vi "SaccadeAnalyser - Main.vi"(8 "error in (no error)":errorcluster, 11 "Data IN":T3={"Impulse Positions"=[{"Start"=5471, "End"=5813, "Impulse Plane"=enum."Yaw", "Impulse Direction +ve?"=FALSE, "Time offset"=0, "Amplitude offset"=0.0}, {"Start"=6974, "End"=7325, "Impulse Plane"=enum."Yaw", "Impulse Direction +ve?"=TRUE, "Time offset"=0, "Amplitude offset"=0.0}, {"Start"=7641, "End"=7980, "Impulse Plane"=enum."Yaw", "Impulse Direction +ve?"=FALSE, "Time offset"=0, "Amplitude offset"=0.0}, {"Start"=9060, "End"=9400, "Impulse Plane"=enum."Yaw", "Impulse Direction +ve?"=FALSE, "Time offset"=0, "Amplitude offset"=0.0}, {"Start"=9938, "End"=10282, "Impulse Plane"=enum."Yaw", "Impulse Direction +ve?"=FALSE, "Time offset"=0, "Amplitude offset"=0.0}, {"Start"=10800, "End"=11142, "Impulse Plane"=enum."Yaw", "Impulse Direction +ve?"=FALSE, "Time offset"=0, "Amplitude offset"=0.0}, {"Start"=11602, "End"=11942, "Impulse Plane"=enum."Yaw", "Impulse Direction +ve?"=TRUE, "Time offset"=0, "Amplitude offset"=0.0}, {"Start"=12449, "End"=12790, "Impulse Plane"=enum."Yaw", "Impulse Direction +ve?"=TRUE, "Time offset"=0, "Amplitude offset"=0.0}, {"Start"=13310, "End"=13653, "Impulse Plane"=enum."Yaw", "Impulse Direction +ve?"=TRUE, "Time offset"=0, "Amplitude offset"=0.0}, {"Start"=14191, "End"=14535, "Impulse Plane"=enum."Yaw", "Impulse Direction +ve?"=TRUE, "Time offset"=0, "Amplitude offset"=0.0}, {"Start"=15040, "End"=15380, "Impulse Plane"=enum."Yaw", "Impulse Direction +ve?"=FALSE, "Time offset"=0, "Amplitude offset"=0.0}, {"Start"=16780, "End"=17124, "Impulse Plane"=enum."Yaw", "Impulse Direction +ve?"=TRUE, "Time offset"=0, "Amplitude offset"=0.0}, {"Start"=17572, "End"=17913, "Impulse Plane"=enum."Yaw", "Impulse Direction +ve?"=FALSE, "Time offset"=0, "Amplitude offset"=0.0}, {"Start"=18369, "End"=18713, "Impulse Plane"=enum."Yaw", "Impulse Direction +ve?"=FALSE, "Time offset"=0, "Amplitude offset"=0.0}, {"Start"=19174, "End"=19519, "Impulse Plane"=enum."Yaw", "Impulse Direction +ve?"=FALSE, "Time offset"=0, "Amplitude offset"=0.0}, {"Start"=19928, "End"=20270, "Impulse Plane"=enum."Yaw", "Impulse Direction +ve?"=TRUE, "Time offset"=0, "Amplitude offset"=0.0}, {"Start"=20762, "End"=21121, "Impulse Plane"=enum."Yaw", "Impulse Direction +ve?"=FALSE, "Time offset"=0, "Amplitude offset"=0.0}, {"Start"=21554, "End"=21888, "Impulse Plane"=enum."Yaw", "Impulse Direction +ve?"=FALSE, "Time offset"=0, "Amplitude offset"=0.0}, {"Start"=22293, "End"=22639, "Impulse Plane"=enum."Yaw", "Impulse Direction +ve?"=TRUE, "Time offset"=0, "Amplitude offset"=0.0}, {"Start"=23109, "End"=23464, "Impulse Plane"=enum."Yaw", "Impulse Direction +ve?"=TRUE, "Time offset"=0, "Amplitude offset"=0.0}, {"Start"=23868, "End"=24215, "Impulse Plane"=enum."Yaw", "Impulse Direction +ve?"=TRUE, "Time offset"=0, "Amplitude offset"=0.0}, {"Start"=24643, "End"=24992, "Impulse Plane"=enum."Yaw", "Impulse Direction +ve?"=FALSE, "Time offset"=0, "Amplitude offset"=0.0}, {"Start"=25685, "End"=26023, "Impulse Plane"=enum."Yaw", "Impulse Direction +ve?"=FALSE, "Time offset"=0, "Amplitude offset"=0.0}, {"Start"=26431, "End"=26768, "Impulse Plane"=enum."Yaw", "Impulse Direction +ve?"=FALSE, "Time offset"=0, "Amplitude offset"=0.0}, {"Start"=27251, "End"=27595, "Impulse Plane"=enum."Yaw", "Impulse Direction +ve?"=FALSE, "Time offset"=0, "Amplitude offset"=0.0}, {"Start"=28832, "End"=29180, "Impulse Plane"=enum."Yaw", "Impulse Direction +ve?"=TRUE, "Time offset"=0, "Amplitude offset"=0.0}, {"Start"=31028, "End"=31383, "Impulse Plane"=enum."LARP", "Impulse Direction +ve?"=FALSE, "Time offset"=0, "Amplitude offset"=0.0}, {"Start"=32603, "End"=32936, "Impulse Plane"=enum."LARP", "Impulse Direction +ve?"=TRUE, "Time offset"=0, "Amplitude offset"=0.0}, {"Start"=33445, "End"=33779, "Impulse Plane"=enum."LARP", "Impulse Direction +ve?"=TRUE, "Time offset"=0, "Amplitude offset"=0.0}, {"Start"=34276, "End"=34629, "Impulse Plane"=enum."LARP", "Impulse Direction +ve?"=FALSE, "Time offset"=0, "Amplitude offset"=0.0}, {"Start"=35114, "End"=35460, "Impulse Plane"=enum."LARP", "Impulse Direction +ve?"=FALSE, "Time offset"=0, "Amplitude offset"=0.0}, {"Start"=35981, "End"=36324, "Impulse Plane"=enum."LARP", "Impulse Direction +ve?"=TRUE, "Time offset"=0, "Amplitude offset"=0.0}, {"Start"=36920, "End"=37249, "Impulse Plane"=enum."LARP", "Impulse Direction +ve?"=TRUE, "Time offset"=0, "Amplitude offset"=0.0}, {"Start"=37988, "End"=38322, "Impulse Plane"=enum."LARP", "Impulse Direction +ve?"=TRUE, "Time offset"=0, "Amplitude offset"=0.0}, {"Start"=38964, "End"=39324, "Impulse Plane"=enum."LARP", "Impulse Direction +ve?"=FALSE, "Time offset"=0, "Amplitude offset"=0.0}, {"Start"=39948, "End"=40284, "Impulse Plane"=enum."LARP", "Impulse Direction +ve?"=TRUE, "Time offset"=0, "Amplitude offset"=0.0}, {"Start"=40958, "End"=41293, "Impulse Plane"=enum."LARP", "Impulse Direction +ve?"=TRUE, "Time offset"=0, "Amplitude offset"=0.0}, {"Start"=41899, "End"=42229, "Impulse Plane"=enum."LARP", "Impulse Direction +ve?"=TRUE, "Time offset"=0, "Amplitude offset"=0.0}, {"Start"=42801, "End"=43154, "Impulse Plane"=enum."LARP", "Impulse Direction +ve?"=FALSE, "Time offset"=0, "Amplitude offset"=0.0}, {"Start"=43641, "End"=43980, "Impulse Plane"=enum."LARP", "Impulse Direction +ve?"=TRUE, "Time offset"=0, "Amplitude offset"=0.0}, {"Start"=44466, "End"=44821, "Impulse Plane"=enum."LARP", "Impulse Direction +ve?"=FALSE, "Time offset"=0, "Amplitude offset"=0.0}, {"Start"=45388, "End"=45722, "Impulse Plane"=enum."LARP", "Impulse Direction +ve?"=TRUE, "Time offset"=0, "Amplitude offset"=0.0}, {"Start"=46149, "End"=46510, "Impulse Plane"=enum."LARP", "Impulse Direction +ve?"=FALSE, "Time offset"=0, "Amplitude offset"=0.0}, {"Start"=47874, "End"=48206, "Impulse Plane"=enum."LARP", "Impulse Direction +ve?"=TRUE, "Time offset"=0, "Amplitude offset"=0.0}, {"Start"=50143, "End"=50479, "Impulse Plane"=enum."RALP", "Impulse Direction +ve?"=TRUE, "Time offset"=0, "Amplitude offset"=0.0}, {"Start"=50976, "End"=51310, "Impulse Plane"=enum."RALP", "Impulse Direction +ve?"=FALSE, "Time offset"=0, "Amplitude offset"=0.0}, {"Start"=51892, "End"=52226, "Impulse Plane"=enum."RALP", "Impulse Direction +ve?"=FALSE, "Time offset"=0, "Amplitude offset"=0.0}, {"Start"=52839, "End"=53171, "Impulse Plane"=enum."RALP", "Impulse Direction +ve?"=FALSE, "Time offset"=0, "Amplitude offset"=0.0}, {"Start"=53676, "End"=54012, "Impulse Plane"=enum."RALP", "Impulse Direction +ve?"=TRUE, "Time offset"=0, "Amplitude offset"=0.0}, {"Start"=54530, "End"=54877, "Impulse Plane"=enum."RALP", "Impulse Direction +ve?"=FALSE, "Time offset"=0, "Amplitude offset"=0.0}, {"Start"=55371, "End"=55711, "Impulse Plane"=enum."RALP", "Impulse Direction +ve?"=TRUE, "Time offset"=0, "Amplitude offset"=0.0}, {"Start"=56153, "End"=56482, "Impulse Plane"=enum."RALP", "Impulse Direction +ve?"=FALSE, "Time offset"=0, "Amplitude offset"=0.0}, {"Start"=57053, "End"=57390, "Impulse Plane"=enum."RALP", "Impulse Direction +ve?"=FALSE, "Time offset"=0, "Amplitude offset"=0.0}, {"Start"=57954, "End"=58292, "Impulse Plane"=enum."RALP", "Impulse Direction +ve?"=FALSE, "Time offset"=0, "Amplitude offset"=0.0}, {"Start"=58794, "End"=59130, "Impulse Plane"=enum."RALP", "Impulse Direction +ve?"=TRUE, "Time offset"=0, "Amplitude offset"=0.0}, {"Start"=59587, "End"=59931, "Impulse Plane"=enum."RALP", "Impulse Direction +ve?"=TRUE, "Time offset"=0, "Amplitude offset"=0.0}, {"Start"=60399, "End"=60744, "Impulse Plane"=enum."RALP", "Impulse Direction +ve?"=FALSE, "Time offset"=0, "Amplitude offset"=0.0}, {"Start"=61218, "End"=61559, "Impulse Plane"=enum."RALP", "Impulse Direction +ve?"=FALSE, "Time offset"=0, "Amplitude offset"=0.0}, {"Start"=62100, "End"=62442, "Impulse Plane"=enum."RALP", "Impulse Direction +ve?"=FALSE, "Time offset"=0, "Amplitude offset"=0.0}, {"Start"=62989, "End"=63322, "Impulse Plane"=enum."RALP", "Impulse Direction +ve?"=FALSE, "Time offset"=0, "Amplitude offset"=0.0}, {"Start"=63787, "End"=64136, "Impulse Plane"=enum."RALP", "Impulse Direction +ve?"=TRUE, "Time offset"=0, "Amplitude offset"=0.0}, {"Start"=64603, "End"=64953, "Impulse Plane"=enum."RALP", "Impulse Direction +ve?"=FALSE, "Time offset"=0, "Amplitude offset"=0.0}, {"Start"=65462, "End"=65795, "Impulse Plane"=enum."RALP", "Impulse Direction +ve?"=FALSE, "Time offset"=0, "Amplitude offset"=0.0}, {"Start"=66308, "End"=66645, "Impulse Plane"=enum."RALP", "Impulse Direction +ve?"=FALSE, "Time offset"=0, "Amplitude offset"=0.0}, {"Start"=67052, "End"=67402, "Impulse Plane"=enum."RALP", "Impulse Direction +ve?"=TRUE, "Time offset"=0, "Amplitude offset"=0.0}], "No. Imp"=15, "Parameter Time Series"=[{"time offset"=0.0, "Offset"=0.0, "Gain"=1.0, "inverse"=FALSE, "filter data"=FALSE, "dots"=FALSE, "interpolate"=FALSE, "List 1"=5, "Color Box"=6618880, "Boolean"=TRUE}, {"time offset"=0.0, "Offset"=0.0, "Gain"=1.0, "inverse"=FALSE, "filter data"=FALSE, "dots"=FALSE, "interpolate"=FALSE, "List 1"=6, "Color Box"=6618880, "Boolean"=FALSE}, {"time offset"=0.0, "Offset"=0.0, "Gain"=1.0, "inverse"=FALSE, "filter data"=FALSE, "dots"=FALSE, "interpolate"=FALSE, "List 1"=7, "Color Box"=6618880, "Boolean"=FALSE}, {"time offset"=0.0, "Offset"=0.0, "Gain"=1.0, "inverse"=FALSE, "filter data"=FALSE, "dots"=FALSE, "interpolate"=FALSE, "List 1"=13, "Color Box"=16777224, "Boolean"=TRUE}, {"time offset"=0.0, "Offset"=0.0, "Gain"=1.0, "inverse"=FALSE, "filter data"=FALSE, "dots"=FALSE, "interpolate"=FALSE, "List 1"=14, "Color Box"=16777224, "Boolean"=FALSE}, {"time offset"=0.0, "Offset"=0.0, "Gain"=1.0, "inverse"=FALSE, "filter data"=FALSE, "dots"=FALSE, "interpolate"=FALSE, "List 1"=15, "Color Box"=16777224, "Boolean"=FALSE}], "Parameter Impuls Series"=[{"Color"=6618880, "Visible"=TRUE, "Channel"=1, "Invert"=FALSE, "Desaccade"=FALSE, "Offset"=0.0, "Gain"=1.0}, {"Color"=6618880, "Visible"=FALSE, "Channel"=6, "Invert"=FALSE, "Desaccade"=FALSE, "Offset"=0.0, "Gain"=1.0}, {"Color"=6618880, "Visible"=FALSE, "Channel"=7, "Invert"=FALSE, "Desaccade"=FALSE, "Offset"=0.0, "Gain"=1.0}, {"Color"=16777224, "Visible"=TRUE, "Channel"=13, "Invert"=FALSE, "Desaccade"=FALSE, "Offset"=0.0, "Gain"=1.0}, {"Color"=16777224, "Visible"=FALSE, "Channel"=14, "Invert"=FALSE, "Desaccade"=FALSE, "Offset"=0.0, "Gain"=1.0}, {"Color"=16777224, "Visible"=FALSE, "Channel"=15, "Invert"=FALSE, "Desaccade"=FALSE, "Offset"=0.0, "Gain"=1.0}], "Experiment Parameters"={"Freq"=0.0, "Vel"=0, "Acc"=0, "Stimulus"="Head Impulse"}, "Autosort File"=refnum, "Data File"={"Data Channels"=array34x71049[2415666 elements], "Sample Rate"=500, "Channel List"=["Hz Position-in-Head", "Hz Velocity-in-Head", "Hy Position-in-Head", "Hy Velocity-in-Head", "Hx Position-in-Head", "Hx Velocity-in-Head", "Hl Velocity-in-Head", "Hr Velocity-in-Head", "Lx Position-in-Head", "Ly Position-in-Head", "Lz Position-in-Head", "Lx Velocity-in-Head", "Ly Velocity-in-Head", "Lz Velocity-in-Head", "Ll Velocity-in-Head", "Lr Velocity-in-Head", "Rx Position-in-Head", "Ry Position-in-Head", "Rz Position-in-Head", "Rx Velocity-in-Head", "Ry Velocity-in-Head", "Rz Velocity-in-Head", "Rl Velocity-in-Head", "Rr Velocity-in-Head", "Target on/off", "aux input 1", "aux input 2", " ", "", "", "", "Target Hor", "Target Ver", ""]}, "Experiment data path"=path "C:/Users/w.figtree/Desktop/Coils Data/3", "Image data path"=path "/Macintosh HD/Users/patrick/Studium/Diploma Thesis/Data Analysis", "LVS data path"=path "/Macintosh HD/Users/patrick/Studium/Diploma Thesis/Data Analysis", "Raw copy path"=path "/Macintosh HD/Users/patrick/Studium/Diploma Thesis/Data Analysis", "filename"="passive_lvs.lvs", "desaccading parameters"={"Tolerance"=3, "Acc Range"=7000.0, "Sample Rate"=500, "Impulse Plane 2"=enum."Yaw", "Impulse dir"=FALSE}, "Experiment Parameters 2"={"Subject"="SE Trial Short Term", "Strain"="", "Rotation plane"="", "Experimenter"=" ", "Trial"=0.0, "Time"=0.0}, "Excel"={"Excel._Application"=refnum, "Use Excel"=TRUE, "Worksheet SINE"=refnum, "Row SINE"=0, "Worksheet TRANS"=refnum, "Row TRANS"=0}, "Session Config File"=refnum, "Autosort Parameter Set"=4, "EMA Version"="EMA 2016a", "desacc "={"Threshold 1 [Acc]"=7000.0, "Threshold 2 [% of TH1]"=60, "tolerance"=3, "Search WD "=0.1, " always use TH2"=FALSE, "Range"=3.0, "Max time"=120.0, "Min time"=20.0, "Velocity Threshold"=150}, "Cycle Nr for Saccades"={"POS"=0, "NEG"=0}, "calibration name"="u_calibration_1_p00001s001_calib.mat", "Excel"=refnum} {"Parameter Time Series"."time offset" format="%.3f"; "Parameter Time Series"."Gain" format="%.1f"; "Parameter Time Series"."Offset" format="%.1f"; "Parameter Time Series"."List 1" items=["Motor-Pos", "Motor-Vel", "Lx Position-in-Head", "Ly Position-in-Head", "Lz Position-in-Head", "Lx Velocity-in-Head", "Ly Velocity-in-Head", "Lz Velocity-in-Head", "Ll Velocity-in-Head", "Lr Velocity-in-Head", "Lx Accel-in-Head", "Ly Accel-in-Head", "Lz Accel-in-Head", "Rx Position-in-Head", "Ry Position-in-Head", "Rz Position-in-Head", "Rx Velocity-in-Head", "Ry Velocity-in-Head", "Rz Velocity-in-Head", "Rl Velocity-in-Head", "Rr Velocity-in-Head", "Rx Accel-in-Head", "Ry Accel-in-Head", "Rz Accel-in-Head", "Global Trigger", "", "", ""]; "Parameter Impuls Series"."Gain" format="%.1f"; "Parameter Impuls Series"."Offset" format="%.1f"}) -> (0 "error out":errorcluster, 3 "Data OUT":T3={"Impulse Positions"=[{"Start"=5471, "End"=5813, "Impulse Plane"=enum."Yaw", "Impulse Direction +ve?"=FALSE, "Time offset"=0, "Amplitude offset"=0.0}, {"Start"=6974, "End"=7325, "Impulse Plane"=enum."Yaw", "Impulse Direction +ve?"=TRUE, "Time offset"=0, "Amplitude offset"=0.0}, {"Start"=7641, "End"=7980, "Impulse Plane"=enum."Yaw", "Impulse Direction +ve?"=FALSE, "Time offset"=0, "Amplitude offset"=0.0}, {"Start"=9060, "End"=9400, "Impulse Plane"=enum."Yaw", "Impulse Direction +ve?"=FALSE, "Time offset"=0, "Amplitude offset"=0.0}, {"Start"=9938, "End"=10282, "Impulse Plane"=enum."Yaw", "Impulse Direction +ve?"=FALSE, "Time offset"=0, "Amplitude offset"=0.0}, {"Start"=10800, "End"=11142, "Impulse Plane"=enum."Yaw", "Impulse Direction +ve?"=FALSE, "Time offset"=0, "Amplitude offset"=0.0}, {"Start"=11602, "End"=11942, "Impulse Plane"=enum."Yaw", "Impulse Direction +ve?"=TRUE, "Time offset"=0, "Amplitude offset"=0.0}, {"Start"=12449, "End"=12790, "Impulse Plane"=enum."Yaw", "Impulse Direction +ve?"=TRUE, "Time offset"=0, "Amplitude offset"=0.0}, {"Start"=13310, "End"=13653, "Impulse Plane"=enum."Yaw", "Impulse Direction +ve?"=TRUE, "Time offset"=0, "Amplitude offset"=0.0}, {"Start"=14191, "End"=14535, "Impulse Plane"=enum."Yaw", "Impulse Direction +ve?"=TRUE, "Time offset"=0, "Amplitude offset"=0.0}, {"Start"=15040, "End"=15380, "Impulse Plane"=enum."Yaw", "Impulse Direction +ve?"=FALSE, "Time offset"=0, "Amplitude offset"=0.0}, {"Start"=16780, "End"=17124, "Impulse Plane"=enum."Yaw", "Impulse Direction +ve?"=TRUE, "Time offset"=0, "Amplitude offset"=0.0}, {"Start"=17572, "End"=17913, "Impulse Plane"=enum."Yaw", "Impulse Direction +ve?"=FALSE, "Time offset"=0, "Amplitude offset"=0.0}, {"Start"=18369, "End"=18713, "Impulse Plane"=enum."Yaw", "Impulse Direction +ve?"=FALSE, "Time offset"=0, "Amplitude offset"=0.0}, {"Start"=19174, "End"=19519, "Impulse Plane"=enum."Yaw", "Impulse Direction +ve?"=FALSE, "Time offset"=0, "Amplitude offset"=0.0}, {"Start"=19928, "End"=20270, "Impulse Plane"=enum."Yaw", "Impulse Direction +ve?"=TRUE, "Time offset"=0, "Amplitude offset"=0.0}, {"Start"=20762, "End"=21121, "Impulse Plane"=enum."Yaw", "Impulse Direction +ve?"=FALSE, "Time offset"=0, "Amplitude offset"=0.0}, {"Start"=21554, "End"=21888, "Impulse Plane"=enum."Yaw", "Impulse Direction +ve?"=FALSE, "Time offset"=0, "Amplitude offset"=0.0}, {"Start"=22293, "End"=22639, "Impulse Plane"=enum."Yaw", "Impulse Direction +ve?"=TRUE, "Time offset"=0, "Amplitude offset"=0.0}, {"Start"=23109, "End"=23464, "Impulse Plane"=enum."Yaw", "Impulse Direction +ve?"=TRUE, "Time offset"=0, "Amplitude offset"=0.0}, {"Start"=23868, "End"=24215, "Impulse Plane"=enum."Yaw", "Impulse Direction +ve?"=TRUE, "Time offset"=0, "Amplitude offset"=0.0}, {"Start"=24643, "End"=24992, "Impulse Plane"=enum."Yaw", "Impulse Direction +ve?"=FALSE, "Time offset"=0, "Amplitude offset"=0.0}, {"Start"=25685, "End"=26023, "Impulse Plane"=enum."Yaw", "Impulse Direction +ve?"=FALSE, "Time offset"=0, "Amplitude offset"=0.0}, {"Start"=26431, "End"=26768, "Impulse Plane"=enum."Yaw", "Impulse Direction +ve?"=FALSE, "Time offset"=0, "Amplitude offset"=0.0}, {"Start"=27251, "End"=27595, "Impulse Plane"=enum."Yaw", "Impulse Direction +ve?"=FALSE, "Time offset"=0, "Amplitude offset"=0.0}, {"Start"=28832, "End"=29180, "Impulse Plane"=enum."Yaw", "Impulse Direction +ve?"=TRUE, "Time offset"=0, "Amplitude offset"=0.0}, {"Start"=31028, "End"=31383, "Impulse Plane"=enum."LARP", "Impulse Direction +ve?"=FALSE, "Time offset"=0, "Amplitude offset"=0.0}, {"Start"=32603, "End"=32936, "Impulse Plane"=enum."LARP", "Impulse Direction +ve?"=TRUE, "Time offset"=0, "Amplitude offset"=0.0}, {"Start"=33445, "End"=33779, "Impulse Plane"=enum."LARP", "Impulse Direction +ve?"=TRUE, "Time offset"=0, "Amplitude offset"=0.0}, {"Start"=34276, "End"=34629, "Impulse Plane"=enum."LARP", "Impulse Direction +ve?"=FALSE, "Time offset"=0, "Amplitude offset"=0.0}, {"Start"=35114, "End"=35460, "Impulse Plane"=enum."LARP", "Impulse Direction +ve?"=FALSE, "Time offset"=0, "Amplitude offset"=0.0}, {"Start"=35981, "End"=36324, "Impulse Plane"=enum."LARP", "Impulse Direction +ve?"=TRUE, "Time offset"=0, "Amplitude offset"=0.0}, {"Start"=36920, "End"=37249, "Impulse Plane"=enum."LARP", "Impulse Direction +ve?"=TRUE, "Time offset"=0, "Amplitude offset"=0.0}, {"Start"=37988, "End"=38322, "Impulse Plane"=enum."LARP", "Impulse Direction +ve?"=TRUE, "Time offset"=0, "Amplitude offset"=0.0}, {"Start"=38964, "End"=39324, "Impulse Plane"=enum."LARP", "Impulse Direction +ve?"=FALSE, "Time offset"=0, "Amplitude offset"=0.0}, {"Start"=39948, "End"=40284, "Impulse Plane"=enum."LARP", "Impulse Direction +ve?"=TRUE, "Time offset"=0, "Amplitude offset"=0.0}, {"Start"=40958, "End"=41293, "Impulse Plane"=enum."LARP", "Impulse Direction +ve?"=TRUE, "Time offset"=0, "Amplitude offset"=0.0}, {"Start"=41899, "End"=42229, "Impulse Plane"=enum."LARP", "Impulse Direction +ve?"=TRUE, "Time offset"=0, "Amplitude offset"=0.0}, {"Start"=42801, "End"=43154, "Impulse Plane"=enum."LARP", "Impulse Direction +ve?"=FALSE, "Time offset"=0, "Amplitude offset"=0.0}, {"Start"=43641, "End"=43980, "Impulse Plane"=enum."LARP", "Impulse Direction +ve?"=TRUE, "Time offset"=0, "Amplitude offset"=0.0}, {"Start"=44466, "End"=44821, "Impulse Plane"=enum."LARP", "Impulse Direction +ve?"=FALSE, "Time offset"=0, "Amplitude offset"=0.0}, {"Start"=45388, "End"=45722, "Impulse Plane"=enum."LARP", "Impulse Direction +ve?"=TRUE, "Time offset"=0, "Amplitude offset"=0.0}, {"Start"=46149, "End"=46510, "Impulse Plane"=enum."LARP", "Impulse Direction +ve?"=FALSE, "Time offset"=0, "Amplitude offset"=0.0}, {"Start"=47874, "End"=48206, "Impulse Plane"=enum."LARP", "Impulse Direction +ve?"=TRUE, "Time offset"=0, "Amplitude offset"=0.0}, {"Start"=50143, "End"=50479, "Impulse Plane"=enum."RALP", "Impulse Direction +ve?"=TRUE, "Time offset"=0, "Amplitude offset"=0.0}, {"Start"=50976, "End"=51310, "Impulse Plane"=enum."RALP", "Impulse Direction +ve?"=FALSE, "Time offset"=0, "Amplitude offset"=0.0}, {"Start"=51892, "End"=52226, "Impulse Plane"=enum."RALP", "Impulse Direction +ve?"=FALSE, "Time offset"=0, "Amplitude offset"=0.0}, {"Start"=52839, "End"=53171, "Impulse Plane"=enum."RALP", "Impulse Direction +ve?"=FALSE, "Time offset"=0, "Amplitude offset"=0.0}, {"Start"=53676, "End"=54012, "Impulse Plane"=enum."RALP", "Impulse Direction +ve?"=TRUE, "Time offset"=0, "Amplitude offset"=0.0}, {"Start"=54530, "End"=54877, "Impulse Plane"=enum."RALP", "Impulse Direction +ve?"=FALSE, "Time offset"=0, "Amplitude offset"=0.0}, {"Start"=55371, "End"=55711, "Impulse Plane"=enum."RALP", "Impulse Direction +ve?"=TRUE, "Time offset"=0, "Amplitude offset"=0.0}, {"Start" (continued)
104.00000000000001, 106.0, 108.0, 110.0, 112.0, 114.0, 116.0, 118.00000000000001, 120.0, 122.0, 124.0, 126.0, 128.0, 130.0, 132.0, 134.0, 136.0, 138.0, 140.0, 142.00000000000003, 144.00000000000003, 146.0, 148.0, 150.0, 152.0, 154.0, 156.0, 158.0, 160.0, 162.0, 164.0, 166.0, 168.0, 170.0, 172.0, 174.00000000000003, 176.0, 178.0, 180.0, 182.0, 184.0, 186.0, 188.0, 190.0, 192.0, 194.0, 196.0, 198.0, 200.0, 202.0, 204.00000000000003, 206.00000000000003, 208.00000000000003, 210.0, 212.0, 214.0, 216.0, 218.0, 220.0, 222.0, 224.0, 226.0, 228.0, 230.0, 232.0, 234.0, 236.00000000000003, 238.00000000000003, 240.0, 242.0, 244.0, 246.0, 248.0, 250.0, 252.0, 254.0, 256.0, 258.0, 260.0, 262.0, 264.0, 266.0, 268.0, 270.0, 272.0, 274.0, 276.0, 278.0, 280.0, 282.0, 284.00000000000006, 286.00000000000006, 288.00000000000006, 290.0, 292.0, 294.0, 296.0, 298.0, 300.0, 302.0, 304.0, 306.0, 308.0, 310.0, 312.0, 314.0, 316.0, 318.0, 320.0, 322.0, 324.0, 326.0, 328.0, 330.0, 332.0, 334.0, 336.0, 338.0, 340.0, 342.0, 344.0, 346.00000000000006, 348.00000000000006, 350.00000000000006, 352.0, 354.0, 356.0, 358.0, 360.0, 362.0, 364.0, 366.0, 368.0, 370.0, 372.0, 374.0, 376.0, 378.0, 380.0, 382.0, 384.0, 386.0, 388.0, 390.0, 392.0, 394.0, 396.0, 398.0, 400.0, 402.0, 404.0, 406.0, 408.00000000000006, 410.00000000000006, 412.00000000000006, 414.00000000000006, 416.00000000000006, 418.0, 420.0, 422.0, 424.0, 426.0, 428.0, 430.0, 432.0, 434.0, 436.0, 438.0, 440.0, 442.0, 444.0, 446.0, 448.0, 450.0, 452.0, 454.0, 456.0, 458.0, 460.0, 462.0, 464.0, 466.0, 468.0, 470.00000000000006, 472.00000000000006, 474.00000000000006, 476.00000000000006, 478.00000000000006, 480.0, 482.0, 484.0, 486.0, 488.0, 490.0, 492.0, 494.0, 496.0, 498.0, 500.0, 502.0, 504.0, 506.0, 508.0, 510.0, 512.0, 514.0, 516.0, 518.0, 520.0, 522.0, 524.0, 526.0, 528.0, 530.0, 532.0, 534.0, 536.0, 538.0, 540.0, 542.0, 544.0, 546.0, 548.0, 550.0, 552.0, 554.0, 556.0, 558.0, 560.0, 562.0, 564.0, 566.0000000000001, 568.0000000000001, 570.0000000000001, 572.0000000000001, 574.0000000000001, 576.0000000000001, 578.0, 580.0, 582.0, 584.0, 586.0, 588.0, 590.0, 592.0, 594.0, 596.0, 598.0, 600.0, 602.0, 604.0, 606.0, 608.0, 610.0, 612.0, 614.0, 616.0, 618.0, 620.0, 622.0, 624.0, 626.0, 628.0, 630.0, 632.0, 634.0, 636.0, 638.0, 640.0, 642.0, 644.0, 646.0, 648.0, 650.0, 652.0, 654.0, 656.0, 658.0, 660.0, 662.0, 664.0, 666.0, 668.0], [0.04992038201718785, 0.15841417568277905, 0.17858167540149594, 0.15312905238445929, 0.12879273253846435, 0.1386267538312591, 0.19119834871886, 0.26744517118748234, 0.3294694061613903, 0.33604542690323846, 0.26750116445730754, 0.13882756764760273, -0.00457400840335076, -0.08930376240759585, -0.03122544770549318, 0.23626243538025626, 0.7326977878601504, 1.414166028082219, 2.18407302630931, 2.91143092377669, 3.4505976401226643, 3.6807231650130703, 3.538299036917895, 3.0375740961591866, 2.2730290152877277, 1.3923240791589553, 0.572883978458961, -0.015453323814009323, -0.25359029677372646, -0.09697114730811052, 0.41567980525341497, 1.1707413546443597, 2.0010012490946743, 2.7260585284931693, 3.1985829335543183, 3.332956582490871, 3.1222617337603964, 2.63734783762464, 2.0087327672521784, 1.396995356354343, 0.9476382692160676, 0.7553993294950168, 0.8473748527615594, 1.181402058393096, 1.66213162160191, 2.164995642103872, 2.565021706411774, 2.7770579425637756, 2.7777673635849727, 2.6013186150579433, 2.3306813660582852, 2.076819233598228, 1.9481292438628854, 2.016991388073549, 2.2989795669998085, 2.749552100833662, 3.2736328956474297, 3.7499302412652673, 4.060800060130227, 4.125340378912859, 3.9311403507880924, 3.535056197748248, 3.049660186385034, 2.624300893859544, 2.4060875775539285, 2.5093105752294194, 2.993320304677124, 3.848304722717669, 4.996773223397807, 6.318170390599681, 7.688214344644706, 9.003185964170115, 10.196919210919303, 11.260714840565495, 12.2491594060802, 13.258988588333356, 14.398222913355678, 15.763109352234887, 17.41424581629392, 19.365482073801317, 21.586770877674706, 24.015338314877916, 26.582943324362425, 29.244991166590985, 31.999704094019627, 34.89270409467796, 38.013451580925384, 41.4776338903614, 45.39813750442575, 49.86051106407923, 54.8996055102276, 60.487486108843896, 66.54041305150024, 72.92794874389115, 79.49091069527614, 86.0732882383193, 92.54343430335877, 98.81704640232888, 104.86380166453532, 110.69767181947952, 116.36816024047974, 121.93679606634197, 127.44946268816003, 132.91382406412202, 138.29013354077009, 143.49090983609346, 148.39593527181597, 152.87217504466742, 156.79159603077275, 160.06260704130017, 162.64877788792944, 164.5616374633256, 165.8592891901892, 166.6238891626943, 166.93327673497157, 166.84560727192155, 166.3680932814025, 165.45691552757975, 164.02818548071699, 161.96591043080474, 159.16084591883293, 155.5358166070166, 151.06037761889493, 145.77461158069093, 139.7884164622531, 133.25880357201612, 126.36444720474383, 119.2860273986354, 112.17741601561518, 105.1525468650749, 98.28906854847438, 91.62060481380246, 85.14400241893199, 78.84223186193547, 72.69596110254957, 66.67462318862016, 60.74867508111842, 54.90283443323352, 49.126842276315514, 43.417641849534206, 37.78234365969709, 32.24059878511545, 26.836290153038057, 21.634339151746794, 16.701708877871617, 12.103037841181745, 7.896149545815408, 4.1128290788135615, 0.7389662736026011, -2.2694903576020735, -4.9631062834405215, -7.405244086308598, -9.65177273250551, -11.721341930325584, -13.600003955279014, -15.252602221067322, -16.630091323905262, -17.684645898322437, -18.3951576449166, -18.774019507133094, -18.85230364678983, -18.67939872359451, -18.309760473378486, -17.782702973493613, -17.114260366081247, -16.298543546223584, -15.32517813268789, -14.187238566587439, -12.894388212139678, -11.486000357145317, -10.02590465717922, -8.595127553420681, -7.280228618080622, -6.148598180573282, -5.236592749098192, -4.553928778071988, -4.088533383914676, -3.8073230410928036, -3.6630957051259516, -3.6150109657845926, -3.6278390081094547, -3.66903344717268, -3.711385162328716, -3.7175002219534328, -3.638365649322722, -3.4289240476014973, -3.057478585829699, -2.5219742752628402, -1.8586527966781206, -1.1389975609344174, -0.47183019522024927, 0.0051455380020754005, 0.15788917699917693, -0.10050061025888996, -0.7911814548039556, -1.8643562384539165, -3.187405881295393, -4.569498848546866, -5.8139278704619395, -6.7478282463364, -7.253448745420589, -7.307372747595566, -6.984682301078392, -6.435022163171514, -5.849969545435848, -5.425648598324794, -5.325281629094702, -5.63615524890895, -6.352882944462618, -7.384002079740541, -8.559439461424077, -9.668039211518757, -10.503952472324885, -10.908138327541469, -10.803458262192532, -10.209367806756003, -9.24090626674652, -8.080681007005104, -6.944230818795323, -6.037426910342507, -5.506280050693961, -5.404708174170484, -5.685918619423186, -6.21971107762246, -6.82533358689519, -7.309516207965832, -7.517365437937178, -7.366810938149376, -6.847446190723453, -6.027476319138884, -5.037258943036763, -4.021281572243785, -3.106723881663414, -2.3861127603837033, -1.9057193800399248, -1.6641085250296699, -1.6357550842919144, -1.7887182069729657, -2.0797865669803848, -2.4613784430723564, -2.87931328602323, -3.2829278591162554, -3.6399358176747985, -3.930540590692001, -4.185841440412954, -4.519901384583601, -5.112600094423929, -6.179934257207675, -7.911857897301076, -10.380842296632798, -13.456630338729223, -16.750182623917276, -19.63301571121884, -21.335243781207225, -21.081763915218374, -18.2841175327463, -12.734024178915037, -4.708677229533636, 5.018081046184022, 15.273118953586463, 24.69383865631704, 31.990547165492487, 36.19894847480768, 36.8668944349022, 34.13346741147935, 28.680271923098346, 21.551397571814505, 13.9200326044393, 6.853263681311434, 1.109113748113744, -2.9572638183698965, -5.386063683488901, -6.525260094996831, -6.873361693133134, -6.913364973447512, -6.977914337377552, -7.176035360345667, -7.398600739376963, -7.3767525082011804, -6.7782328355304795, -5.314655641339901, -2.8256467063059447, 0.6726090248953283, 4.98148672460113, 9.750320796626117, 14.530187559033408, 18.84255920678958, 22.26067541171979, 24.468305768199688, 25.29294718130975, 24.725614427990152, 22.9030335665933, 20.082655608922238, 16.606151876437476, 12.82963888753322, 9.079726996951507, 5.622531347536689, 2.6217090367480265, 0.13171202491932155, -1.8838458215461478, -3.5233802618856194, -4.91150074028557, -6.173130009585858, -7.408881055173729, -8.664646778406222, -9.92458311171681, -11.12491778059621, -12.164256102990326, -12.926429930262247, -13.308922541262364, -13.239115051984019, -12.688617129803168, -11.680068508276396, -10.28596817566143, -8.619076823723638, -6.8072801732139006, -4.977472566204141, -3.2450998627929843, -1.699500663571817, -0.39723303554407496, 0.6456925599396672, 1.4455339547691926, 2.023868943252673, 2.40182753031554, 2.597658890354133, 2.615611688992259, 2.4512690594426902, 2.097642800762138, 1.5504992618844369, 0.8296317099263332, -0.011760473109973524, -0.898827295135341, -1.7432784721434178, -2.455414534839041]}, {[0.0, 2.0, 4.0, 6.0, 8.0, 10.0, 12.0, 14.0, 16.0, 18.000000000000004, 20.0, 22.0, 24.0, 26.000000000000004, 28.0, 30.0, 32.0, 34.0, 36.00000000000001, 38.0, 40.0, 42.0, 44.0, 46.0, 48.0, 50.0, 52.00000000000001, 54.0, 56.0, 58.0, 60.0, 62.0, 64.0, 66.0, 68.0, 70.0, 72.00000000000001, 74.0, 76.0, 78.0, 80.0, 82.0, 84.0, 86.0, 88.0, 90.0, 92.0, 94.0, 96.0, 98.0, 100.0, 102.00000000000001, 104.00000000000001, 106.0, 108.0, 110.0, 112.0, 114.0, 116.0, 118.00000000000001, 120.0, 122.0, 124.0, 126.0, 128.0, 130.0, 132.0, 134.0, 136.0, 138.0, 140.0, 142.00000000000003, 144.00000000000003, 146.0, 148.0, 150.0, 152.0, 154.0, 156.0, 158.0, 160.0, 162.0, 164.0, 166.0, 168.0, 170.0, 172.0, 174.00000000000003, 176.0, 178.0, 180.0, 182.0, 184.0, 186.0, 188.0, 190.0, 192.0, 194.0, 196.0, 198.0, 200.0, 202.0, 204.00000000000003, 206.00000000000003, 208.00000000000003, 210.0, 212.0, 214.0, 216.0, 218.0, 220.0, 222.0, 224.0, 226.0, 228.0, 230.0, 232.0, 234.0, 236.00000000000003, 238.00000000000003, 240.0, 242.0, 244.0, 246.0, 248.0, 250.0, 252.0, 254.0, 256.0, 258.0, 260.0, 262.0, 264.0, 266.0, 268.0, 270.0, 272.0, 274.0, 276.0, 278.0, 280.0, 282.0, 284.00000000000006, 286.00000000000006, 288.00000000000006, 290.0, 292.0, 294.0, 296.0, 298.0, 300.0, 302.0, 304.0, 306.0, 308.0, 310.0, 312.0, 314.0, 316.0, 318.0, 320.0, 322.0, 324.0, 326.0, 328.0, 330.0, 332.0, 334.0, 336.0, 338.0, 340.0, 342.0, 344.0, 346.00000000000006, 348.00000000000006, 350.00000000000006, 352.0, 354.0, 356.0, 358.0, 360.0, 362.0, 364.0, 366.0, 368.0, 370.0, 372.0, 374.0, 376.0, 378.0, 380.0, 382.0, 384.0, 386.0, 388.0, 390.0, 392.0, 394.0, 396.0, 398.0, 400.0, 402.0, 404.0, 406.0, 408.00000000000006, 410.00000000000006, 412.00000000000006, 414.00000000000006, 416.00000000000006, 418.0, 420.0, 422.0, 424.0, 426.0, 428.0, 430.0, 432.0, 434.0, 436.0, 438.0, 440.0, 442.0, 444.0, 446.0, 448.0, 450.0, 452.0, 454.0, 456.0, 458.0, 460.0, 462.0, 464.0, 466.0, 468.0, 470.00000000000006, 472.00000000000006, 474.00000000000006, 476.00000000000006, 478.00000000000006, 480.0, 482.0, 484.0, 486.0, 488.0, 490.0, 492.0, 494.0, 496.0, 498.0, 500.0, 502.0, 504.0, 506.0, 508.0, 510.0, 512.0, 514.0, 516.0, 518.0, 520.0, 522.0, 524.0, 526.0, 528.0, 530.0, 532.0, 534.0, 536.0, 538.0, 540.0, 542.0, 544.0, 546.0, 548.0, 550.0, 552.0, 554.0, 556.0, 558.0, 560.0, 562.0, 564.0, 566.0000000000001, 568.0000000000001, 570.0000000000001, 572.0000000000001, 574.0000000000001, 576.0000000000001, 578.0, 580.0, 582.0, 584.0, 586.0, 588.0, 590.0, 592.0, 594.0, 596.0, 598.0, 600.0, 602.0, 604.0, 606.0, 608.0, 610.0, 612.0, 614.0, 616.0, 618.0, 620.0, 622.0, 624.0, 626.0, 628.0, 630.0, 632.0, 634.0, 636.0, 638.0, 640.0, 642.0, 644.0, 646.0, 648.0, 650.0, 652.0, 654.0, 656.0, 658.0, 660.0, 662.0, 664.0, 666.0, 668.0], [0.06811297872756228, 0.01707691464348393, -0.0029316795212057656, -0.018371635138466402, -0.0542419341462157, -0.12324447550139972, -0.21981306669672707, -0.3191162631877944, -0.3853854038940563, -0.3843579085985379, -0.30437797985139503, -0.1664789665300923, -0.017769334490307376, 0.06862919302039172, 0.013104685658458237, -0.24114913861073983, -0.709333253854556, -1.351598990540456, -2.075622182814767, -2.753071542994334, -3.246216629685337, -3.443449967376811, -3.286367039037831, -2.791374332901265, -2.051529141203167, -1.2105609505019466, -0.4403291048291216, 0.09601987150864488, 0.28620327185831584, 0.0919344247244478, -0.4423285837620785, -1.1989490655453743, -2.009497024906068, -2.6945611442154345, -3.1102502224856075, -3.1773935367996238, -2.898039897130179, -2.353443274375975, -1.684014162208868, -1.0575586797480234, -0.622984378715925, -0.47347998056239504, -0.6266828095259971, -1.0270679039930393, -1.5690220717276038, -2.1190951404570306, -2.54956813966023, -2.779552448106653, -2.7895908254476565, -2.618860676067743, -2.352435864524903, -2.093848698492252, -1.9367005319072188, -1.9373752595012403, -2.103354399108734, -2.399366287498072, -2.7620015653891814, -3.1211357852220005, -3.4186287524182504, -3.6236871208071846, -3.7450535834045713, -3.817946376182001, -3.8859888168671204, -3.9913068551006026, -4.157735245453354, -4.388591325996881, -4.6732363152460525, -4.994493297578687, -5.337310207009276, -5.702737161776087, -6.121366746488304, -6.643068076473353, -7.320282018360008, -8.205626664881649, -9.342663338610144, -10.751802729833212, -12.428003541980054, -14.3403029147095, -16.440257730359697, -18.674757629156378, -20.993764005443836, -23.36094550703045, -25.766167573394647, -28.235984867149952, -30.83064641351026, -33.63339995706863, -36.745311701228715, -40.27040505521088, -44.29407874919056, -48.870946189857676, -54.00959526902649, -59.663906206975355, -65.7386581494263, -72.09737120363829, -78.58246030020933, -85.0352581421007, -91.3134523513386, -97.31362354068435, -102.97527187162223, -108.28408268059235, -113.26702471639702, -117.96733172180792, -122.42684847414944, -126.66981282582509, -130.68989907667182, -134.44283460888644, -137.85244951870885, -140.82165420094103, -143.24223062902917, -145.02170566485017, -146.1037912555284, -146.46968334697482, -146.1471196893165, -145.20629627467477, -143.74220064879705, -141.85872825081555, -139.64370902034784, -137.15798008041577, -134.42257527977037, -131.4126853108042, -128.08076518877618, -124.36618833100033, -120.20643043471809, -115.56964072369297, -110.4603120398877, -104.91662067262685, -99.01459414696029, -92.84879592980549, -86.51455625875208, -80.10405919393807, -73.69570633615069, -67.34436860943498, -61.079868879950936, -54.91881846904339, -48.8738566758385, -42.94324202006271, -37.12579137611928, -31.43575468987897, -25.893713973831275, -20.529814577915463, -15.378567619948482, -10.475762977646728, -5.87078036515235, -1.6138072100983745, 2.2589012438241216, 5.719319198016697, 8.753394056833748, 11.371987432326065, 13.614850118136234, 15.53086899295791, 17.16306402142841, 18.55930505462024, 19.75481537637341, 20.749089170347897, 21.515467519080165, 22.01484738199841, 22.199541133152387, 22.028741064356986, 21.491661564892, 20.609113930182346, 19.428716656693503, 18.02788467843449, 16.500143833663433, 14.930160091602048, 13.376483906376627, 11.87036794903375, 10.415710880119065, 8.989572465999547, 7.560845831193208, 6.1027325862580595, 4.603048893552675, 3.07753895294191, 1.570133296299682, 0.13842686919653385, -1.1568119174650138, -2.2602235619324857, -3.131991953285361, -3.75399476360169, -4.133526753166105, -4.2962023287540525, -4.2844484046818785, -4.151852782862191, -3.94982606172549, -3.729759679211063, -3.5434807457679414, -3.4278343586013795, -3.4010361304890293, -3.460941924695227, -3.5813444726372614, -3.7158673293531495, -3.797382732606872, -3.7457232909032574, -3.4878987015258818, -2.976388065807112, -2.2012372945460585, -1.2013567070120303, -0.06614869140339244, 1.0827569045557948, 2.1216308405257394, 2.941114971981066, 3.465146635393052, 3.6810319703878003, 3.6416994052849176, 3.447348103262948, 3.225317286944987, 3.104267279621971, 3.184616011120855, 3.5156161941209936, 4.0871040504899945, 4.827929362851712, 5.614676731384651, 6.299894275922779, 6.745370728633619, 6.84967349681979, 6.570829842117675, 5.943921524319785, 5.072323900665897, 4.108133393451007, 3.229933838105311, 2.5947631747208058, 2.30455203873153, 2.3874723862129703, 2.790268295892536, 3.3952890667926305, 4.043416410085843, 4.567698519208367, 4.839138058302615, 4.791625214237972, 4.422629524254613, 3.795701022726382, 3.0201197776996414, 2.2145862641113117, 1.4836841728016847, 0.8988987524946157, 0.49280070366187473, 0.26672795826633355, 0.20414573750868892, 0.28833816851917715, 0.5097965758076993, 0.8647418104989528, 1.3410934015396394, 1.9109823952853278, 2.52580516764164, 3.1028997180898754, 3.5431869478949656, 3.757219828036531, 3.687889855685584, 3.335312780011749, 2.7646912248993374, 2.0965982164565182, 1.4797263793432553, 1.0477012265478458, 0.8908774199349385, 1.0438705295470805, 1.4696667413133204, 2.071543882617245, 2.7270146458245303, 3.319160693464326, 3.7638053025332354, 4.022366364599833, 4.096422395061614, 4.0183552557659725, 3.839385525911659, 3.606770845134818, 3.3522729511422367, 3.0969910212666183, 2.85630743125981, 2.6457056931852394, 2.4847926333426593, 2.394220979675119, 2.385816103160016, 2.454403411404333, 2.5815312358312417, 2.7383786341780136, 2.8874618436135493, 2.996881486307256, 3.051711492335385, 3.0601475608858513, 3.053380776250896, 3.067708340558502, 3.1274342906317205, 3.234457056908898, 3.36211169923049, 3.4591239557532933, 3.466689294427814, 3.3429106085475917, 3.0792966880165826, 2.709342310081312, 2.3079129249876114, 1.9720181453804109, 1.796923585982143, 1.8581080803733132, 2.17728877460085, 2.7130702250324816, 3.3838043305668988, 4.070707388743466, 4.644883381909614, 5.0073945947340235, 5.1000437236075875, 4.9126499987834205, 4.48347140592128, 3.8831852409382375, 3.1986454349252043, 2.519243710829821, 1.9165205342500835, 1.4331658384077302, 1.0847603527471747, 0.8636811848461314, 0.7492308632821785, 0.7164782241651273, 0.7406704091576592, 0.8071249548709076, 0.9134990728194428, 1.0649594396912203, 1.271952277018636, 1.5391030784550257, 1.8564719934987681, 2.1983658293373436, 2.5222255077429394, 2.772647991591127, 2.887869721810326, 2.811259754156945, 2.514732326295733, 2.012414201142896, 1.3577577685336109, 0.6407542736655927, -0.025039157128084355, -0.5255953523570946, -0.7603567392766966, -0.668844351205168, -0.25610992848806813, 0.4173561284864338, 1.246890852854512, 2.100085066130018]}, {[0.0, 2.0, 4.0, 6.0, 8.0, 10.0, 12.0, 14.0, 16.0, 18.000000000000004, 20.0, 22.0, 24.0, 26.000000000000004, 28.0, 30.0, 32.0, 34.0, 36.00000000000001, 38.0, 40.0, 42.0, 44.0, 46.0, 48.0, 50.0, 52.00000000000001, 54.0, 56.0, 58.0, 60.0, 62.0, 64.0, 66.0, 68.0, 70.0, 72.00000000000001, 74.0, 76.0, 78.0, 80.0, 82.0, 84.0, 86.0, 88.0, 90.0, 92.0, 94.0, 96.0, 98.0, 100.0, 102.00000000000001, 104.00000000000001, 106.0, 108.0, 110.0, 112.0, 114.0, 116.0, 118.00000000000001, 120.0, 122.0, 124.0, 126.0, 128.0, 130.0, 132.0, 134.0, 136.0, 138.0, 140.0, 142.00000000000003, 144.00000000000003, 146.0, 148.0, 150.0, 152.0, 154.0, 156.0, 158.0, 160.0, 162.0, 164.0, 166.0, 168.0, 170.0, 172.0, 174.00000000000003, 176.0, 178.0, 180.0, 182.0, 184.0, 186.0, 188.0, 190.0, 192.0, 194.0, 196.0, 198.0, 200.0, 202.0, 204.00000000000003, 206.00000000000003, 208.00000000000003, 210.0, 212.0, 214.0, 216.0, 218.0, 220.0, 222.0, 224.0, 226.0, 228.0, 230.0, 232.0, 234.0, 236.00000000000003, 238.00000000000003, 240.0, 242.0, 244.0, 246.0, 248.0, 250.0, 252.0, 254.0, 256.0, 258.0, 260.0, 262.0, 264.0, 266.0, 268.0, 270.0, 272.0, 274.0, 276.0, 278.0, 280.0, 282.0, 284.00000000000006, 286.00000000000006, 288.00000000000006, 290.0, 292.0, 294.0, 296.0, 298.0, 300.0, 302.0, 304.0, 306.0, 308.0, 310.0, 312.0, 314.0, 316.0, 318.0, 320.0, 322.0, 324.0, 326.0, 328.0, 330.0, 332.0, 334.0, 336.0, 338.0, 340.0, 342.0, 344.0, 346.00000000000006, 